vi "FlexMag - 24-03-2023.vi"() -> ()   [LabVIEW 2018] (continued)
  # "LN2 CONTROL"
  # "Click on buttons to start LN2 flow. Use during the deposition."
  # "CH4"
  # "CH3"
  # "CH2"
  # "CH1"
  # "Water Bypass"
  # "Water sensors might be fail. To by pass water check, please activate this button. Hereby, it will check only main flow."
  # "Process List"
  # "Current Recipe Number :"
  # "System Status"
  # "System Warnings"
  # "Technical Service"
  # "CC"
  # "SoV"
  # "BG BV"
  # "Set Value"
  # "sccm"
  # "Actual Value"
  # "sccm"
  # "%"
  # "Set Position"
  # "Actual Position"
  # "%"
  # "Set Pressure"
  # "mbar"
  # "Baratron Pressure"
  # "mbar"
  # "Set Forward Power :"
  # "Watt"
  # "RF Net Power         :"
  # "Watt"
  # "RF Bias                  :"
  # "Volt"
  # "sec"
  # "sec"
  # "sec"
  # "sec"
  # "CH3 Magnetron"
  # "CC"
  # "BG BV"
  # "SoV"
  # "Set Value"
  # "sccm"
  # "Actual Value"
  # "sccm"
  # "Set Position"
  # "%"
  # "Actual Position"
  # "%"
  # "Set Pressure"
  # "mbar"
  # "Baratron Pressure"
  # "mbar"
  # "Set DC Power"
  # "watt"
  # "Actual DC Power"
  # "watt"
  # "Actual DC Voltage"
  # "volts"
  # "Ramp Up Time"
  # "sec"
  # "Ramp Down Time"
  # "sec"
  # "CH2 Magnetron"
  # "CC"
  # "BG BV"
  # "SoV"
  # "Set Value"
  # "sccm"
  # "Actual Value"
  # "sccm"
  # "%"
  # "Set Position"
  # "%"
  # "Actual Position"
  # "Set Pressure"
  # "mbar"
  # "Baratron Pressure"
  # "mbar"
  # "Set DC Power"
  # "watt"
  # "Actual DC Power"
  # "watt"
  # "Actual DC Voltage"
  # "volts"
  # "Ramp Up Time"
  # "sec"
  # "Ramp Down Time"
  # "sec"
  # "SoV"
  # "CC"
  # "BG BV"
  # "Set Value"
  # "sccm"
  # "Actual Value"
  # "sccm"
  # "%"
  # "Set Position"
  # "%"
  # "Actual Position"
  # "Set Pressure"
  # "mbar"
  # "Baratron Pressure"
  # "mbar"
  # "Microwave 1 Power"
  # "watt"
  # "Microwave 2 Power"
  # "watt"
  # "2-3"
  # "1-2"
  # "2-3"
  # "2-1"
  # "3-2"
  # "4-3"
  # "Final Output Voltage"
  # "Volts"
  # "Lap Number R Target"
  # "lap"
  # "Total Target"
  # "cm"
  # "Final Right Diameter"
  # "mm"
  # "rpm"
  # "Min Circular Speed"
  # "Max Circular Speed"
  # "rpm"
  # "Initial Output Voltage"
  # "Volts"
  # "Decreasing Voltage"
  # "Volts"
  # "Current Voltage"
  # "Volts"
  # "Initial Right Diameter"
  # "mm"
  # "Web Thickness"
  # "µm"
  # "Web Speed"
  # "cm/min"
  # "Target Interval"
  # "cm"
  # "Lap Number L Target"
  # "lap"
  # "Actual Freq."
  # "f"
  # "Step Number 2"
  # "QR Scanner off sec :"
  # "PL VBV"
  # "BG BV"
  # "CH VBV"
  # "TP BV"
  # "CC"
  # "PC GV"
  # "TRNS BP LEFT"
  # "CH1-CH2 TRNS"
  # "MP"
  # "TP"
  # "BG BV"
  # "PL VBV"
  # "CH VBV"
  # "TP BV"
  # "CC"
  # "TRNS BP LEFT"
  # "TRNS BP RIGHT"
  # "PC GV"
  # "CH1-CH2 TRNS"
  # "CH2-CH3 TRNS"
  # "TP"
  # "MP"
  # "PL VBV"
  # "BG BV"
  # "CH VBV"
  # "CC"
  # "TP BV"
  # "TRNS BP LEFT"
  # "TRNS BP RIGHT"
  # "PC GV"
  # "CH2-CH3 TRNS"
  # "CH3-CH4 TRNS"
  # "TP"
  # "MP"
  # "BG BV"
  # "PL VBV"
  # "CH VBV"
  # "CC"
  # "TP BV"
  # "PC GV"
  # "CH3-CH4 TRNS"
  # "TRNS BP RIGHT"
  # "TP"
  # "MP"
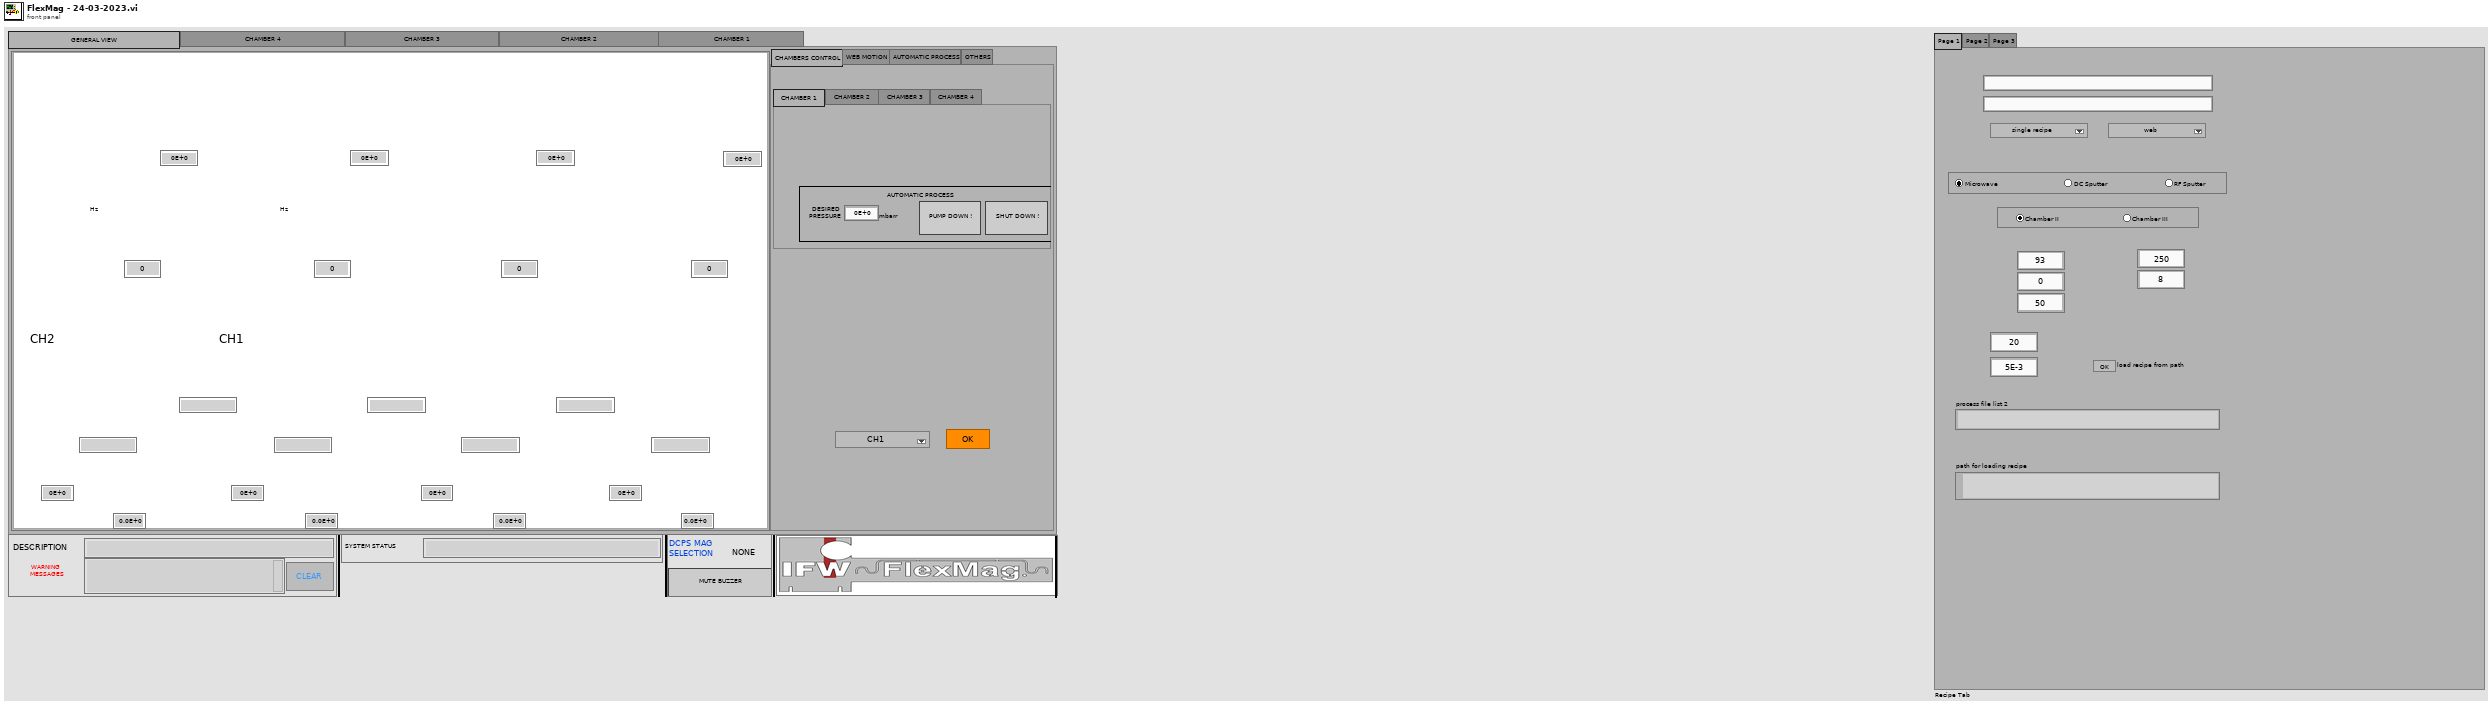
[diagram p1: front panel]
types:
  T1 = enum32{"GENERAL VIEW                                                                     ", "CHAMBER 4                                                                      ", "CHAMBER 3                                                                ", "CHAMBER 2                                                                   ", "CHAMBER 1                                                           "}
  T2 = enum32{"CHAMBERS CONTROL", "WEB MOTION", "AUTOMATIC PROCESS", "OTHERS"}
  T3 = enum32{"CHAMBER 1     ", "CHAMBER 2      ", "CHAMBER 3     ", "CHAMBER 4     "}
  T4 = enum32{"RF Power Supply Control", "  Ramp Timer", "Pulsing ", "Capacitor"}
  T5 = enum32{"CENTER MOXAs", "CH1 MOXAs", "CH2 MOXAs", "CH3 MOXAs", "CH4 MOXAs", "COM PORTs", "DCPS", "RFPS", "MICROWAVE", "Timers", "Safety", "Paths", "Pfeiffer Turbo Pump", "Vat pcgv", "Counter", "Pressures", "Auto process", "CH1-2 pd-sd leds", "CH3-4 pd-sd leds", "MFCs control", "LN2 control", "LN2 control 2", "GUI&JPEG", "TRANSFER", "Rolling", "Recipe Files", "Auto Deposition", "QR Scanner", "gui buttons", "Keysight"}
  T6 = enum32{"MOXA1", "MOXA2", "MOXA3", "MOXA4", "MOXA5", "MOXA6"}
  T7 = enum32{"Page 1", "Page 2", "Page 3", "Page 4", "Page 5"}
  T8 = cluster{"proportional gain (Kc)":dbl, "integral time (Ti, min)":dbl, "derivative time (Td, min)":dbl}
  T9 = enum32{"CH1-Microwave", "CH2-DCPS", "CH3-DCPS", "CH4-RFPS"}
  T10 = typedef "imagedata.ctl" = cluster{"image type":i32, "image depth":i32, "image":u8[], "mask":u8[], "colors":u32[], "Rectangle":cluster{"left":i16, "top":i16, "right":i16, "bottom":i16}}
  T11 = enum16{"User-specified Font", "Application Font", "System Font", "Dialog Font"}
  T12 = cluster{"Font Name:":string, "Size":i16, "Strikeout?":bool, "Italic?":bool, "Underline?":bool, "Outline?":bool, "Shadow?":bool, "Bold?":bool}
  T13 = enum8{"Enabled", "Disabled", "Disabled and Grayed Out"}
  T14 = typedef "LVMouseTypeDef.ctl" = cluster{"Mouse Position":cluster{"X":i32, "Y":i32}, "Mouse Modifiers":cluster{"Button Down":bool, "Shift Mod":bool, "Menu Mod":bool, "Option Mod":bool}}
  T15 = cluster{"Mode":enum16{"RTU", "ASCII"}, "Slave Address":u8}
  T16 = enum16{"open", "replace", "create", "open or create", "replace or create", "replace or create with confirmation"}
  T17 = cluster{"final output voltage":dbl, "final output voltage":dbl}
  T18 = cluster{"initial output voltage":dbl, "final output voltage":dbl}
diagram:
  w1 = TRUE ("dep. for?")
  (unwired) refnum<visa-resource-name> "USB0::0x0957::0x1807::MY59080144::INSTR" ("counter 2")
  w14 = FALSE
  w19 = TRUE ("Tp4_stop_cmnd")
  w30 = FALSE
  w31 = "OPEN !" ("ch1_door_open")
  w37 = u16 0 items=["None", "Odd", "Even", "Mark", "Space"] ("Parity")
  w47 = u16 0 items=["None", "Odd", "Even", "Mark", "Space"] ("Parity")
  w88 = 5e-05 ("ch1 desired pressure")
  w86 = FALSE ("Visible")
  w110 = u16 0 items=["None", "Odd", "Even", "Mark", "Space"] ("Parity")
  w117 = u16 0 items=["None", "Odd", "Even", "Mark", "Space"] ("Parity")
  w128 = u16 0 items=["None", "Odd", "Even", "Mark", "Space"] ("Parity")
  w139 = u16 0 items=["None", "Odd", "Even", "Mark", "Space"] ("Parity")
  w146 = u16 0 items=["None", "Odd", "Even", "Mark", "Space"] ("Parity")
  # "*important notes*\n\nchambers pressures should be checked\n to open trns bp bv"
  # "DO 1&2"
  n1 = flat-sequence {
    frame #0 {
      # "CH4"
      # "CH3"
      # "CH2"
      # "chamber 1 front main screen"
      # "CH1"
      # "Trns-GV-Bp-Left"
      # "Trns-GV-Bp-Right"
      # "Trns-GV"
      # "CH-Atm"
      # "BG-BV"
      # "BG"
      # "CH-CC"
      # "CH-PG"
      # "Pc-gv"
      # "Tp"
      # "Tp-vbv"
      # "Tp-bv"
      # "Pl-PG"
      # "Pl-atm"
      # "Pl-vbv"
      # "Mp"
      n2 = disable-structure shown="Disabled" {
        disable-tunnel: "path to JPEG file" -> [w331 _]
        frame Disabled {
          n3 = Build Path(base path=w331, name or relative path="trns gv front left on.jpg") -> (appended path=w363:path)
          n4 = Build Path(base path=w331, name or relative path="trns gv front left fail.jpg") -> (appended path=w360:path)
          n5 = Build Path(base path=w331, name or relative path="trns gv front right on.jpg") -> (appended path=w352:path)
          n6 = Build Path(base path=w331, name or relative path="trns gv top right on.jpg") -> (appended path=w351:path)
          n7 = Build Path(base path=w331, name or relative path="trns gv front right fail.jpg") -> (appended path=w355:path)
          n8 = Build Path(base path=w331, name or relative path="trns gv top right fail.jpg") -> (appended path=w348:path)
          n9 = Build Path(base path=w331, name or relative path="trns gv top left on.jpg") -> (appended path=w332:path)
          n10 = Build Path(base path=w331, name or relative path="trns gv top left fail.jpg") -> (appended path=w335:path)
          n11 = call <vilib>:"Read JPEG File.vi"("path to JPEG file"=w363) -> ("image data"=w359:T10)  [unwired: 8 in, 2 out]
          n12 = call <vilib>:"Read JPEG File.vi"("path to JPEG file"=w360) -> ("image data"=w362:T10)  [unwired: 8 in, 2 out]
          n13 = call <vilib>:"Read JPEG File.vi"("path to JPEG file"=w352) -> ("image data"=w356:T10)  [unwired: 8 in, 2 out]
          n14 = call <vilib>:"Read JPEG File.vi"("path to JPEG file"=w351) -> ("image data"=w347:T10)  [unwired: 8 in, 2 out]
          n15 = call <vilib>:"Read JPEG File.vi"("path to JPEG file"=w355) -> ("image data"=w353:T10)  [unwired: 8 in, 2 out]
          n16 = call <vilib>:"Read JPEG File.vi"("path to JPEG file"=w348) -> ("image data"=w350:T10)  [unwired: 8 in, 2 out]
          n17 = call <vilib>:"Read JPEG File.vi"("path to JPEG file"=w332) -> ("image data"=w336:T10)  [unwired: 8 in, 2 out]
          n18 = call <vilib>:"Read JPEG File.vi"("path to JPEG file"=w335) -> ("image data"=w333:T10)  [unwired: 8 in, 2 out]
          n19 = call <vilib>:"Unflatten Pixmap.vi"("image data"=w359) -> ("24-bit pixmap"=→"trns gv front left on jpeg":u32[][])  [unwired: 4 in, 6 out]
          n20 = call <vilib>:"Unflatten Pixmap.vi"("image data"=w362) -> ("24-bit pixmap"=→"trns gv front left fail jpeg":u32[][])  [unwired: 4 in, 6 out]
          n21 = call <vilib>:"Unflatten Pixmap.vi"("image data"=w356) -> ("24-bit pixmap"=→"trns gv front right on jpeg":u32[][])  [unwired: 4 in, 6 out]
          n22 = call <vilib>:"Unflatten Pixmap.vi"("image data"=w353) -> ("24-bit pixmap"=→"trns gv front right fail jpeg":u32[][])  [unwired: 4 in, 6 out]
          n23 = call <vilib>:"Unflatten Pixmap.vi"("image data"=w347) -> ("24-bit pixmap"=→"trns gv top right on  jpeg":u32[][])  [unwired: 4 in, 6 out]
          n24 = call <vilib>:"Unflatten Pixmap.vi"("image data"=w350) -> ("24-bit pixmap"=→"trns gv top right fail jpeg":u32[][])  [unwired: 4 in, 6 out]
          n25 = call <vilib>:"Unflatten Pixmap.vi"("image data"=w336) -> ("24-bit pixmap"=→"trns gv top left on jpeg":u32[][])  [unwired: 4 in, 6 out]
          n26 = call <vilib>:"Unflatten Pixmap.vi"("image data"=w333) -> ("24-bit pixmap"=→"trns gv top left fail jpeg":u32[][])  [unwired: 4 in, 6 out]
        }
        frame Enabled {
        }
      }
      n27 = Build Path(base path="path to JPEG file", name or relative path="vbv on.jpg") -> (appended path=w316:path)
      n28 = Build Path(base path="path to JPEG file", name or relative path="main screen.jpg") -> (appended path=w330:path)
      n29 = Build Path(base path="path to JPEG file", name or relative path="vbv fail.jpg") -> (appended path=w319:path)
      n30 = Build Path(base path="path to JPEG file", name or relative path="mp on.jpg") -> (appended path=w325:path)
      n31 = Build Path(base path="path to JPEG file", name or relative path="mp fail.jpg") -> (appended path=w322:path)
      n32 = Build Path(base path="path to JPEG file", name or relative path="trns gv bp bv left on.jpg") -> (appended path=w197:path)
      n33 = Build Path(base path="path to JPEG file", name or relative path="trns gv bp bv left fail.jpg") -> (appended path=w200:path)
      n34 = Build Path(base path="path to JPEG file", name or relative path="pl atm on.jpg") -> (appended path=w315:path)
      n35 = Build Path(base path="path to JPEG file", name or relative path="trns gv bp bv right on.jpg") -> (appended path=w208:path)
      n36 = Build Path(base path="path to JPEG file", name or relative path="pl atm fail.jpg") -> (appended path=w312:path)
      n37 = Build Path(base path="path to JPEG file", name or relative path="gv on.jpg") -> (appended path=w213:path)
      n38 = Build Path(base path="path to JPEG file", name or relative path="trns gv bp bv right fail.jpg") -> (appended path=w205:path)
      n39 = Build Path(base path="path to JPEG file", name or relative path="gv fail.jpg") -> (appended path=w216:path)
      n40 = Build Path(base path="path to JPEG file", name or relative path="pl pg on.jpg") -> (appended path=w304:path)
      n41 = Build Path(base path="path to JPEG file", name or relative path="pl pg fail.jpg") -> (appended path=w307:path)
      n42 = Build Path(base path="path to JPEG file", name or relative path="ch atm on.jpg") -> (appended path=w226:path)
      n43 = Build Path(base path="path to JPEG file", name or relative path="ch atm fail.jpg") -> (appended path=w223:path)
      n44 = Build Path(base path="path to JPEG file", name or relative path="bg on.jpg") -> (appended path=w242:path)
      n45 = Build Path(base path="path to JPEG file", name or relative path="cc on.jpg") -> (appended path=w243:path)
      n46 = Build Path(base path="path to JPEG file", name or relative path="bg fail.jpg") -> (appended path=w239:path)
      n47 = Build Path(base path="path to JPEG file", name or relative path="cc fail.jpg") -> (appended path=w246:path)
      n48 = Build Path(base path="path to JPEG file", name or relative path="tp on.jpg") -> (appended path=w286:path)
      n49 = Build Path(base path="path to JPEG file", name or relative path="ch pg on.jpg") -> (appended path=w276:path)
      n50 = Build Path(base path="path to JPEG file", name or relative path="bg bv on.jpg") -> (appended path=w227:path)
      n51 = Build Path(base path="path to JPEG file", name or relative path="tp bv on.jpg") -> (appended path=w303:path)
      n52 = Build Path(base path="path to JPEG file", name or relative path="tp fail.jpg") -> (appended path=w289:path)
      n53 = Build Path(base path="path to JPEG file", name or relative path="ch pg fail.jpg") -> (appended path=w273:path)
      n54 = Build Path(base path="path to JPEG file", name or relative path="bg bv fail.jpg") -> (appended path=w230:path)
      n55 = Build Path(base path="path to JPEG file", name or relative path="tp bv fail.jpg") -> (appended path=w300:path)
      n56 = Build Path(base path="path to JPEG file", name or relative path="tp vbv on.jpg") -> (appended path=w292:path)
      n57 = Build Path(base path="path to JPEG file", name or relative path="tp vbv fail.jpg") -> (appended path=w295:path)
      n58 = Build Path(base path="path to JPEG file", name or relative path="pc gv middle.jpg") -> (appended path=w277:path)
      n59 = Build Path(base path="path to JPEG file", name or relative path="pc gv on.jpg") -> (appended path=w285:path)
      n60 = Build Path(base path="path to JPEG file", name or relative path="pc gv fail.jpg") -> (appended path=w282:path)
      n61 = Build Path(base path="path to JPEG file", name or relative path="chamber 4 top main screen.jpg") -> (appended path=w178:path)
      n62 = Build Path(base path="path to JPEG file", name or relative path="chamber 2 top main screen.jpg") -> (appended path=w179:path)
      n63 = Build Path(base path="path to JPEG file", name or relative path="chamber 4 front main screen.jpg") -> (appended path=w175:path)
      n64 = Build Path(base path="path to JPEG file", name or relative path="chamber 2 front main screen.jpg") -> (appended path=w182:path)
      n65 = Build Path(base path="path to JPEG file", name or relative path="chamber 2 top main screen.jpg") -> (appended path=w163:path)
      n66 = Build Path(base path="path to JPEG file", name or relative path="sov on.jpg") -> (appended path=w157:path)
      n67 = Build Path(base path="path to JPEG file", name or relative path="chamber 1 top main screen.jpg") -> (appended path=w194:path)
      n68 = Build Path(base path="path to JPEG file", name or relative path="chamber 2 front main screen.jpg") -> (appended path=w166:path)
      n69 = Build Path(base path="path to JPEG file", name or relative path="sov fail.jpg") -> (appended path=w159:path)
      n70 = Build Path(base path="path to JPEG file", name or relative path="chamber 1 front main screen.jpg") -> (appended path=w191:path)
      n71 = call <vilib>:"Read JPEG File.vi"("path to JPEG file"=w316) -> ("image data"=w318:T10)  [unwired: 8 in, 2 out]
      n72 = call <vilib>:"Read JPEG File.vi"("path to JPEG file"=w330) -> ("image data"=w328:T10)  [unwired: 8 in, 2 out]
      n73 = call <vilib>:"Read JPEG File.vi"("path to JPEG file"=w319) -> ("image data"=w321:T10)  [unwired: 8 in, 2 out]
      n74 = call <vilib>:"Read JPEG File.vi"("path to JPEG file"=w325) -> ("image data"=w327:T10)  [unwired: 8 in, 2 out]
      n75 = Build Path(base path="path to JPEG file", name or relative path="araba.jpg") -> (appended path=w154:path)
      n76 = call <vilib>:"Read JPEG File.vi"("path to JPEG file"=w322) -> ("image data"=w324:T10)  [unwired: 8 in, 2 out]
      n77 = call <vilib>:"Read JPEG File.vi"("path to JPEG file"=w197) -> ("image data"=w201:T10)  [unwired: 8 in, 2 out]
      n78 = call <vilib>:"Read JPEG File.vi"("path to JPEG file"=w200) -> ("image data"=w198:T10)  [unwired: 8 in, 2 out]
      n79 = call <vilib>:"Read JPEG File.vi"("path to JPEG file"=w315) -> ("image data"=w313:T10)  [unwired: 8 in, 2 out]
      n80 = call <vilib>:"Read JPEG File.vi"("path to JPEG file"=w208) -> ("image data"=w204:T10)  [unwired: 8 in, 2 out]
      n81 = call <vilib>:"Read JPEG File.vi"("path to JPEG file"=w312) -> ("image data"=w310:T10)  [unwired: 8 in, 2 out]
      n82 = call <vilib>:"Read JPEG File.vi"("path to JPEG file"=w213) -> ("image data"=w217:T10)  [unwired: 8 in, 2 out]
      n83 = call <vilib>:"Read JPEG File.vi"("path to JPEG file"=w205) -> ("image data"=w207:T10)  [unwired: 8 in, 2 out]
      n84 = call <vilib>:"Read JPEG File.vi"("path to JPEG file"=w216) -> ("image data"=w214:T10)  [unwired: 8 in, 2 out]
      n85 = call <vilib>:"Read JPEG File.vi"("path to JPEG file"=w304) -> ("image data"=w306:T10)  [unwired: 8 in, 2 out]
      n86 = call <vilib>:"Read JPEG File.vi"("path to JPEG file"=w307) -> ("image data"=w309:T10)  [unwired: 8 in, 2 out]
      n87 = call <vilib>:"Read JPEG File.vi"("path to JPEG file"=w226) -> ("image data"=w222:T10)  [unwired: 8 in, 2 out]
      n88 = call <vilib>:"Read JPEG File.vi"("path to JPEG file"=w223) -> ("image data"=w225:T10)  [unwired: 8 in, 2 out]
      n89 = call <vilib>:"Read JPEG File.vi"("path to JPEG file"=w242) -> ("image data"=w238:T10)  [unwired: 8 in, 2 out]
      n90 = call <vilib>:"Read JPEG File.vi"("path to JPEG file"=w243) -> ("image data"=w247:T10)  [unwired: 8 in, 2 out]
      n91 = call <vilib>:"Read JPEG File.vi"("path to JPEG file"=w239) -> ("image data"=w241:T10)  [unwired: 8 in, 2 out]
      n92 = call <vilib>:"Read JPEG File.vi"("path to JPEG file"=w246) -> ("image data"=w244:T10)  [unwired: 8 in, 2 out]
      n93 = call <vilib>:"Read JPEG File.vi"("path to JPEG file"=w286) -> ("image data"=w290:T10)  [unwired: 8 in, 2 out]
      n94 = call <vilib>:"Read JPEG File.vi"("path to JPEG file"=w276) -> ("image data"=w272:T10)  [unwired: 8 in, 2 out]
      n95 = call <vilib>:"Read JPEG File.vi"("path to JPEG file"=w227) -> ("image data"=w231:T10)  [unwired: 8 in, 2 out]
      n96 = call <vilib>:"Read JPEG File.vi"("path to JPEG file"=w303) -> ("image data"=w301:T10)  [unwired: 8 in, 2 out]
      n97 = call <vilib>:"Read JPEG File.vi"("path to JPEG file"=w289) -> ("image data"=w287:T10)  [unwired: 8 in, 2 out]
      n98 = call <vilib>:"Read JPEG File.vi"("path to JPEG file"=w273) -> ("image data"=w275:T10)  [unwired: 8 in, 2 out]
      n99 = call <vilib>:"Read JPEG File.vi"("path to JPEG file"=w230) -> ("image data"=w228:T10)  [unwired: 8 in, 2 out]
      n100 = call <vilib>:"Read JPEG File.vi"("path to JPEG file"=w300) -> ("image data"=w298:T10)  [unwired: 8 in, 2 out]
      n101 = call <vilib>:"Read JPEG File.vi"("path to JPEG file"=w292) -> ("image data"=w294:T10)  [unwired: 8 in, 2 out]
      n102 = call <vilib>:"Read JPEG File.vi"("path to JPEG file"=w295) -> ("image data"=w297:T10)  [unwired: 8 in, 2 out]
      n103 = call <vilib>:"Read JPEG File.vi"("path to JPEG file"=w277) -> ("image data"=w279:T10)  [unwired: 8 in, 2 out]
      n104 = call <vilib>:"Read JPEG File.vi"("path to JPEG file"=w285) -> ("image data"=w283:T10)  [unwired: 8 in, 2 out]
      n105 = call <vilib>:"Read JPEG File.vi"("path to JPEG file"=w282) -> ("image data"=w280:T10)  [unwired: 8 in, 2 out]
      n106 = call <vilib>:"Read JPEG File.vi"("path to JPEG file"=w178) -> ("image data"=w174:T10)  [unwired: 8 in, 2 out]
      n107 = call <vilib>:"Read JPEG File.vi"("path to JPEG file"=w179) -> ("image data"=w183:T10)  [unwired: 8 in, 2 out]
      n108 = call <vilib>:"Read JPEG File.vi"("path to JPEG file"=w175) -> ("image data"=w177:T10)  [unwired: 8 in, 2 out]
      n109 = call <vilib>:"Read JPEG File.vi"("path to JPEG file"=w182) -> ("image data"=w180:T10)  [unwired: 8 in, 2 out]
      n110 = call <vilib>:"Read JPEG File.vi"("path to JPEG file"=w163) -> ("image data"=w167:T10)  [unwired: 8 in, 2 out]
      n111 = call <vilib>:"Read JPEG File.vi"("path to JPEG file"=w157) -> ("image data"=w160:T10)  [unwired: 8 in, 2 out]
      n112 = call <vilib>:"Read JPEG File.vi"("path to JPEG file"=w194) -> ("image data"=w190:T10)  [unwired: 8 in, 2 out]
      n113 = call <vilib>:"Read JPEG File.vi"("path to JPEG file"=w166) -> ("image data"=w164:T10)  [unwired: 8 in, 2 out]
      n114 = call <vilib>:"Read JPEG File.vi"("path to JPEG file"=w191) -> ("image data"=w193:T10)  [unwired: 8 in, 2 out]
      n115 = call <vilib>:"Read JPEG File.vi"("path to JPEG file"=w159) -> ("image data"=w150:T10)  [unwired: 8 in, 2 out]
      n116 = call <vilib>:"Read JPEG File.vi"("path to JPEG file"=w154) -> ("image data"=w156:T10)  [unwired: 8 in, 2 out]
      n117 = call <vilib>:"Unflatten Pixmap.vi"("image data"=w318) -> ("24-bit pixmap"=→"pl vbv on jpeg":u32[][])  [unwired: 4 in, 6 out]
      n118 = call <vilib>:"Unflatten Pixmap.vi"("image data"=w328) -> ("24-bit pixmap"=→"main screen jpeg":u32[][])  [unwired: 4 in, 6 out]
      n119 = call <vilib>:"Unflatten Pixmap.vi"("image data"=w321) -> ("24-bit pixmap"=→"pl vbv fail jpeg":u32[][])  [unwired: 4 in, 6 out]
      n120 = call <vilib>:"Unflatten Pixmap.vi"("image data"=w327) -> ("24-bit pixmap"=→"mp on jpeg":u32[][])  [unwired: 4 in, 6 out]
      n121 = call <vilib>:"Unflatten Pixmap.vi"("image data"=w324) -> ("24-bit pixmap"=→"mp fail jpeg":u32[][])  [unwired: 4 in, 6 out]
      n122 = call <vilib>:"Unflatten Pixmap.vi"("image data"=w201) -> ("24-bit pixmap"=→"gv bp left on jpeg":u32[][])  [unwired: 4 in, 6 out]
      n123 = call <vilib>:"Unflatten Pixmap.vi"("image data"=w198) -> ("24-bit pixmap"=→"gv bp left fail jpeg":u32[][])  [unwired: 4 in, 6 out]
      n124 = call <vilib>:"Unflatten Pixmap.vi"("image data"=w313) -> ("24-bit pixmap"=→"pl atm on jpeg":u32[][])  [unwired: 4 in, 6 out]
      n125 = call <vilib>:"Unflatten Pixmap.vi"("image data"=w204) -> ("24-bit pixmap"=→"gv bp right on jpeg":u32[][])  [unwired: 4 in, 6 out]
      n126 = call <vilib>:"Unflatten Pixmap.vi"("image data"=w207) -> ("24-bit pixmap"=→"gv bp right fail jpeg":u32[][])  [unwired: 4 in, 6 out]
      n127 = call <vilib>:"Unflatten Pixmap.vi"("image data"=w310) -> ("24-bit pixmap"=→"pl atm fail jpeg":u32[][])  [unwired: 4 in, 6 out]
      n128 = call <vilib>:"Unflatten Pixmap.vi"("image data"=w217) -> ("24-bit pixmap"=→"trns gv on jpeg":u32[][])  [unwired: 4 in, 6 out]
      n129 = call <vilib>:"Unflatten Pixmap.vi"("image data"=w214) -> ("24-bit pixmap"=→"trns gv fail jpeg":u32[][])  [unwired: 4 in, 6 out]
      n130 = call <vilib>:"Unflatten Pixmap.vi"("image data"=w306) -> ("24-bit pixmap"=→"pl pg on jpeg":u32[][])  [unwired: 4 in, 6 out]
      n131 = call <vilib>:"Unflatten Pixmap.vi"("image data"=w309) -> ("24-bit pixmap"=→"pl pg fail jpeg":u32[][])  [unwired: 4 in, 6 out]
      n132 = call <vilib>:"Unflatten Pixmap.vi"("image data"=w222) -> ("24-bit pixmap"=→"ch atm on jpeg":u32[][])  [unwired: 4 in, 6 out]
      n133 = call <vilib>:"Unflatten Pixmap.vi"("image data"=w225) -> ("24-bit pixmap"=→"ch atm fail jpeg":u32[][])  [unwired: 4 in, 6 out]
      n134 = call <vilib>:"Unflatten Pixmap.vi"("image data"=w238) -> ("24-bit pixmap"=→"bg on jpeg":u32[][])  [unwired: 4 in, 6 out]
      n135 = call <vilib>:"Unflatten Pixmap.vi"("image data"=w241) -> ("24-bit pixmap"=→"bg fail jpeg":u32[][])  [unwired: 4 in, 6 out]
      n136 = call <vilib>:"Unflatten Pixmap.vi"("image data"=w247) -> ("24-bit pixmap"=→"cc on jpeg":u32[][])  [unwired: 4 in, 6 out]
      n137 = call <vilib>:"Unflatten Pixmap.vi"("image data"=w244) -> ("24-bit pixmap"=→"cc fail jpeg":u32[][])  [unwired: 4 in, 6 out]
      n138 = call <vilib>:"Unflatten Pixmap.vi"("image data"=w290) -> ("24-bit pixmap"=→"tp start jpeg":u32[][])  [unwired: 4 in, 6 out]
      n139 = call <vilib>:"Unflatten Pixmap.vi"("image data"=w287) -> ("24-bit pixmap"=→"tp fail jpeg":u32[][])  [unwired: 4 in, 6 out]
      n140 = call <vilib>:"Unflatten Pixmap.vi"("image data"=w272) -> ("24-bit pixmap"=→"ch pg on jpeg":u32[][])  [unwired: 4 in, 6 out]
      n141 = call <vilib>:"Unflatten Pixmap.vi"("image data"=w275) -> ("24-bit pixmap"=→"ch pg fail jpeg":u32[][])  [unwired: 4 in, 6 out]
      n142 = call <vilib>:"Unflatten Pixmap.vi"("image data"=w231) -> ("24-bit pixmap"=→"bg bv on jpeg":u32[][])  [unwired: 4 in, 6 out]
      n143 = call <vilib>:"Unflatten Pixmap.vi"("image data"=w228) -> ("24-bit pixmap"=→"bg bv fail jpeg":u32[][])  [unwired: 4 in, 6 out]
      n144 = call <vilib>:"Unflatten Pixmap.vi"("image data"=w301) -> ("24-bit pixmap"=→"tp bv on jpeg":u32[][])  [unwired: 4 in, 6 out]
      n145 = call <vilib>:"Unflatten Pixmap.vi"("image data"=w298) -> ("24-bit pixmap"=→"tp bv fail jpeg":u32[][])  [unwired: 4 in, 6 out]
      n146 = call <vilib>:"Unflatten Pixmap.vi"("image data"=w294) -> ("24-bit pixmap"=→"tp vbv on jpeg":u32[][])  [unwired: 4 in, 6 out]
      n147 = call <vilib>:"Unflatten Pixmap.vi"("image data"=w297) -> ("24-bit pixmap"=→"tp vbv fail jpeg":u32[][])  [unwired: 4 in, 6 out]
      n148 = call <vilib>:"Unflatten Pixmap.vi"("image data"=w279) -> ("24-bit pixmap"=→"pc gv half jpeg":u32[][])  [unwired: 4 in, 6 out]
      n149 = call <vilib>:"Unflatten Pixmap.vi"("image data"=w283) -> ("24-bit pixmap"=→"pc gv on jpeg":u32[][])  [unwired: 4 in, 6 out]
      n150 = call <vilib>:"Unflatten Pixmap.vi"("image data"=w280) -> ("24-bit pixmap"=→"pc gv fail jpeg":u32[][])  [unwired: 4 in, 6 out]
      n151 = call <vilib>:"Unflatten Pixmap.vi"("image data"=w174) -> ("24-bit pixmap"=→"ch4 top main jpeg":u32[][])  [unwired: 4 in, 6 out]
      n152 = call <vilib>:"Unflatten Pixmap.vi"("image data"=w177) -> ("24-bit pixmap"=→"ch4 front main jpeg":u32[][])  [unwired: 4 in, 6 out]
      n153 = call <vilib>:"Unflatten Pixmap.vi"("image data"=w183) -> ("24-bit pixmap"=→"ch2 top main jpeg":u32[][])  [unwired: 4 in, 6 out]
      n154 = call <vilib>:"Unflatten Pixmap.vi"("image data"=w180) -> ("24-bit pixmap"=→"ch2 front main jpeg":u32[][])  [unwired: 4 in, 6 out]
      n155 = call <vilib>:"Unflatten Pixmap.vi"("image data"=w167) -> ("24-bit pixmap"=→"ch3 top main jpeg":u32[][])  [unwired: 4 in, 6 out]
      n156 = call <vilib>:"Unflatten Pixmap.vi"("image data"=w164) -> ("24-bit pixmap"=→"ch3 front main jpeg":u32[][])  [unwired: 4 in, 6 out]
      n157 = call <vilib>:"Unflatten Pixmap.vi"("image data"=w160) -> ("24-bit pixmap"=→"sov on jpeg":u32[][])  [unwired: 4 in, 6 out]
      n158 = call <vilib>:"Unflatten Pixmap.vi"("image data"=w190) -> ("24-bit pixmap"=→"ch1 top main jpeg":u32[][])  [unwired: 4 in, 6 out]
      n159 = call <vilib>:"Unflatten Pixmap.vi"("image data"=w193) -> ("24-bit pixmap"=→"ch1 front main jpeg":u32[][])  [unwired: 4 in, 6 out]
      n160 = call <vilib>:"Unflatten Pixmap.vi"("image data"=w150) -> ("24-bit pixmap"=→"sov fail jpeg":u32[][])  [unwired: 4 in, 6 out]
      n161 = call <vilib>:"Unflatten Pixmap.vi"("image data"=w156) -> ("24-bit pixmap"=→"casette jpeg":u32[][])  [unwired: 4 in, 6 out]
    }
  }
  n162 = stacked-sequence {
    frame #0 {
      n163 = property on="initial cover tab" class="TabCtl (strict)"("Visible"=TRUE) -> ()  [unwired: 2 in, 2 out]
      n164 = Wait (ms)(milliseconds to wait=u32 100) -> ()  [unwired: 1 out]
      "initial string" <- "Please Wait ! System Initializing ..." ("String")
    }
    frame #1 {
      n165 = while {
        i -> [w368]
        stop <- w372 stop-if-true
        n166 = Wait Until Next ms Multiple(millisecond multiple=u32 100) -> ()  [unwired: 1 out]
        n167 = Multiply(x=2 ("y"), y=w368) -> (x*y=w369:i32)
        "Slide" <- w369
        n168 = Greater Or Equal?(x=w369, y=100) -> (x >= y?=w372:bool)
        n169 = Greater Or Equal?(x=w369, y=70) -> (x >= y?=w370:bool)
        n170 = Not(x=w372) -> (.not. x?=w373:bool)
        n171 = case shown="True" w370 {
          frame False {
          }
          frame True {
            n172 = local write "initial string"("Welcome to FlexMag R-2-R Sputter System .." ("initial string")) -> ()
          }
        }
        n173 = property on="initial cover tab" class="TabCtl (strict)"("Visible"=w373) -> ()  [unwired: 2 in, 2 out]
      }
    }
  }
  n174 = while {
    stop <- FALSE stop-if-true
    n175 = stacked-sequence {
      frame #0 {
        n176 = Compound Arithmetic op=OR("cc3 open gui", "cc3 open gui 1", "cc3 open gui 2") -> (w411:bool)
        n177 = Compound Arithmetic op=OR("cc2 close gui", "cc2 close gui 1", "cc2 close gui 2") -> (w400:bool)
        n178 = Compound Arithmetic op=OR("cc3 close gui", "cc3 close gui 1", "cc3 close gui 2") -> (w410:bool)
        n179 = Compound Arithmetic op=OR("cc2 open gui", "cc2 open gui 1", "cc2 open gui 2") -> (w419:bool)
        n180 = Compound Arithmetic op=OR("cc4 close gui", "cc4 close gui 1", "cc4 close gui 2") -> (w406:bool)
        n181 = Compound Arithmetic op=OR("cc1 close gui", "cc1 close gui 1", "cc1 close gui 2") -> (w420:bool)
        n182 = Compound Arithmetic op=OR("cc4 open gui", "cc4 open gui 1", "cc4 open gui 2") -> (w408:bool)
        n183 = Or(x="mp1 start gui", y="mp1 start gui 1") -> (x .or. y?=w570:bool)
        n184 = Or(x="mp2 start gui", y="mp2 start gui 1") -> (x .or. y?=w565:bool)
        n185 = Or(x="mp3 start gui", y="mp3 start gui 1") -> (x .or. y?=w559:bool)
        n186 = Or(x="mp4 start gui", y="mp4 start gui 1") -> (x .or. y?=w562:bool)
        n187 = Or(x="tpbv1 open gui", y="tpbv1 open gui 1") -> (x .or. y?=w503:bool)
        n188 = Or(x="tpbv2 open gui", y="tpbv2 open gui 1") -> (x .or. y?=w506:bool)
        n189 = Or(x="tpbv3 open gui", y="tpbv3 open gui 1") -> (x .or. y?=w510:bool)
        n190 = Or(x="tpbv4 open gui", y="tpbv4 open gui 1") -> (x .or. y?=w507:bool)
        n191 = Or(x="mp1 stop gui", y="mp1 stop gui 1") -> (x .or. y?=w568:bool)
        n192 = Or(x="mp2 stop gui", y="mp2 stop gui 1") -> (x .or. y?=w566:bool)
        n193 = Or(x="mp3 stop gui", y="mp3 stop gui 1") -> (x .or. y?=w560:bool)
        n194 = Or(x="mp4 stop gui", y="mp4 stop gui 1") -> (x .or. y?=w561:bool)
        n195 = Or(x="tpbv1 close gui", y="tpbv1 close gui 1") -> (x .or. y?=w504:bool)
        n196 = Or(x="tpbv2 close gui", y="tpbv2 close gui 1") -> (x .or. y?=w505:bool)
        n197 = Or(x="tpbv3 close gui", y="tpbv3 close gui 1") -> (x .or. y?=w509:bool)
        n198 = Or(x="tpbv4 close gui", y="tpbv4 close gui 1") -> (x .or. y?=w508:bool)
        n199 = Compound Arithmetic op=OR("cc1 open gui", "cc1 open gui 1", "cc1 open gui 2") -> (w422:bool)
        n200 = case shown="True" w400 {
          frame False {
          }
          frame True {
            n201 = local write "CH2_CC_DO"(FALSE ("CH2_MP_DO")) -> ()
          }
        }
        n202 = case shown="True" w411 {
          tunnel: "cc3 open safety" -> [_ w583]
          frame False {
          }
          frame True {
            n203 = case shown="True" w583 {
              frame False {
                n204 = local write "Warning Message"("CH3 CC Cannot be opened !" ("Warning Message")) -> ()
              }
              frame True {
                n205 = local write "CH3_CC_DO"(TRUE ("CH3_MP_DO")) -> ()
              }
            }
          }
        }
        n206 = case shown="True" w410 {
          frame False {
          }
          frame True {
            n207 = local write "CH3_CC_DO"(FALSE ("CH3_MP_DO")) -> ()
          }
        }
        n208 = case shown="True" w408 {
          tunnel: "cc4 open safety" -> [_ w579]
          frame False {
          }
          frame True {
            n209 = case shown="True" w579 {
              frame False {
                n210 = local write "Warning Message"("CH4 CC Cannot be opened !" ("Warning Message")) -> ()
              }
              frame True {
                n211 = local write "CH4_CC_DO"(TRUE ("CH4_MP_DO")) -> ()
              }
            }
          }
        }
        n212 = case shown="True" w406 {
          frame False {
          }
          frame True {
            n213 = local write "CH4_CC_DO"(FALSE ("CH4_MP_DO")) -> ()
          }
        }
        n214 = case shown="True" w422 {
          tunnel: "cc1 open safety" -> [_ w575]
          frame False {
          }
          frame True {
            n215 = case shown="True" w575 {
              frame False {
                n216 = local write "Warning Message"("CH1 CC Cannot be opened !" ("Warning Message")) -> ()
              }
              frame True {
                n217 = local write "CH1_CC_DO"(TRUE ("CH3_MP_DO")) -> ()
              }
            }
          }
        }
        n218 = case shown="True" w420 {
          frame False {
          }
          frame True {
            n219 = local write "CH1_CC_DO"(FALSE ("CH3_MP_DO")) -> ()
          }
        }
        n220 = case shown="True" w419 {
          tunnel: "cc2 open safety" -> [_ w571]
          frame False {
          }
          frame True {
            n221 = case shown="True" w571 {
              frame False {
                n222 = local write "Warning Message"("CH2 CC Cannot be opened !" ("Warning Message")) -> ()
              }
              frame True {
                n223 = local write "CH2_CC_DO"(TRUE ("CH4_MP_DO")) -> ()
              }
            }
          }
        }
        n224 = case shown="True" w570 {
          tunnel: "mp1 start safety" -> [_ w693]
          frame False {
          }
          frame True {
            n225 = case shown="True" w693 {
              frame False {
                n226 = local write "Warning Message"("CH1 MP Cannot be started !" ("Warning Message")) -> ()
              }
              frame True {
                n227 = stacked-sequence {
                  frame #0 {
                    w695 = TRUE ("CH1_PL_ATM_DO")
                    n228 = local write "CH1_PL_ATM_DO"(w695) -> ()
                    n229 = local write "CH1_CH_ATM_DO"(w695) -> ()
                  }
                  frame #1 {
                    n230 = Wait (ms)(milliseconds to wait=u32 500) -> ()  [unwired: 1 out]
                  }
                  frame #2 {
                    n231 = local write "CH1_MP_DO"(TRUE ("CH1_MP_DO")) -> ()
                  }
                }
              }
            }
          }
        }
        n232 = case shown="True" w568 {
          tunnel: "mp1 stop safety" -> [_ w688]
          frame False {
          }
          frame True {
            n233 = case shown="True" w688 {
              frame False {
                n234 = local write "Warning Message"("CH1 MP Cannot be stopped !" ("Warning Message")) -> ()
              }
              frame True {
                n235 = stacked-sequence {
                  frame #0 {
                    w690 = FALSE ("CH1_MP_DO")
                    n236 = local write "CH1_MP_DO"(w690) -> ()
                    n237 = local write "CH1_PL_ATM_DO"(w690) -> ()
                    n238 = local write "CH1_CH_ATM_DO"(w690) -> ()
                  }
                  frame #1 {
                    n239 = Wait (ms)(milliseconds to wait=u32 500) -> ()  [unwired: 1 out]
                  }
                  frame #2 {
                    n240 = local write "CH1_PL_VBV_DO"(TRUE ("CH1_PL_VBV_DO")) -> ()
                  }
                }
              }
            }
          }
        }
        n241 = case shown="True" w565 {
          tunnel: "mp2 start safety" -> [_ w683]
          frame False {
          }
          frame True {
            n242 = case shown="True" w683 {
              frame False {
                n243 = local write "Warning Message"("CH2 MP Cannot be started !" ("Warning Message")) -> ()
              }
              frame True {
                n244 = stacked-sequence {
                  frame #0 {
                    w685 = TRUE ("CH1_PL_ATM_DO")
                    n245 = local write "CH2_PL_ATM_DO"(w685) -> ()
                    n246 = local write "CH2_CH_ATM_DO"(w685) -> ()
                  }
                  frame #1 {
                    n247 = Wait (ms)(milliseconds to wait=u32 500) -> ()  [unwired: 1 out]
                  }
                  frame #2 {
                    n248 = local write "CH2_MP_DO"(TRUE ("CH1_MP_DO")) -> ()
                  }
                }
              }
            }
          }
        }
        n249 = case shown="True" w566 {
          tunnel: "mp2 stop safety" -> [_ w678]
          frame False {
          }
          frame True {
            n250 = case shown="True" w678 {
              frame False {
                n251 = local write "Warning Message"("CH2 MP Cannot be stopped !" ("Warning Message")) -> ()
              }
              frame True {
                n252 = stacked-sequence {
                  frame #0 {
                    w680 = FALSE ("CH2_MP_DO")
                    n253 = local write "CH2_PL_ATM_DO"(w680) -> ()
                    n254 = local write "CH2_CH_ATM_DO"(w680) -> ()
                    n255 = local write "CH2_MP_DO"(w680) -> ()
                  }
                  frame #1 {
                    n256 = Wait (ms)(milliseconds to wait=u32 500) -> ()  [unwired: 1 out]
                  }
                  frame #2 {
                    n257 = local write "CH2_PL_VBV_DO"(TRUE ("CH2_PL_VBV_DO")) -> ()
                  }
                }
              }
            }
          }
        }
        n258 = case shown="True" w559 {
          tunnel: "mp3 start safety" -> [_ w673]
          frame False {
          }
          frame True {
            n259 = case shown="True" w673 {
              frame False {
                n260 = local write "Warning Message"("CH3 MP Cannot be started !" ("Warning Message")) -> ()
              }
              frame True {
                n261 = stacked-sequence {
                  frame #0 {
                    w675 = TRUE ("CH1_PL_ATM_DO")
                    n262 = local write "CH3_PL_ATM_DO"(w675) -> ()
                    n263 = local write "CH3_CH_ATM_DO"(w675) -> ()